vi "UHR-Fleezers Control (host) - 12.8.vi"() -> ()   [LabVIEW 2012] (continued)
              tunnel: w1167 -> [w1171]
              tunnel: w1166 -> [w1170]
              tunnel: w1165 -> [w1169]
              tunnel: w1164 -> [w1168]
              frame #0 {
                n826 = local write "BD 1 Frequency 1 (MHz)"(w1171) -> ()
                n827 = local write "BD 2 Frequency 1 (MHz)"(w1170) -> ()
                n828 = local write "BD 1 Frequency 2 (MHz)"(w1169) -> ()
                n829 = local write "BD 2 Frequency 2 (MHz)"(w1168) -> ()
              }
              frame #1 {
                n830 = property on="Update all trap values" class="Bool (strict)"("Val(Sgnl)"=TRUE ("Value (Signaling)")) -> ()  [unwired: 2 in, 2 out]
              }
            }
          }
        }
      }
      event "Stop All": Value Change {
        # "Stopping blue laser before shutting off program"
        n831 = event-data() -> ()  [unwired: 1 in, 5 out]
        n832 = local read "Delay (ms)"() -> (w1279:i32)
        n833 = call "serial write macro.vi"("String"="l0", "Delay (ms)"=w1279, "VISA resource name"=w1282) -> ("read buffer"=w1277:string, "error out"=w1278:errorcluster, "VISA resource name out"=w1281:refnum<visa-resource-name>)
        n834 = local write "read blue buffer"(w1277) -> ()
        n835 = local write "Blue Error Out"(w1278) -> ()
        n836 = VISA Close(VISA resource name=w1281) -> ()  [unwired: 1 in, 1 out]
        n837 = local read "Stop All"() -> (w1283:bool)
      }
    }
    n838 = node-c288() -> ()  [unwired: 1 in, 1 out]
  }
  n839 = node-c288(2 ("Processor")) -> (w66:T23)  [unwired: 3 out]
  n840 = node-c288() -> (w22:T23)  [unwired: 4 out]
  n841 = node-c288() -> (w68:T23)  [unwired: 4 out]
  n842 = while "Duncan's play event loop" {
    stop <- w1285 stop-if-true
    n843 = Create User Event(user event datatype=TRUE ("Boolean")) -> (user event=w1286:refnum<user-event>)  [unwired: 1 in, 1 out]
    n844 = Create User Event(user event datatype=TRUE ("Boolean")) -> (user event=w1293:refnum<user-event>)  [unwired: 1 in, 1 out]
    n845 = global write "Global for fluorescence simulation mean (30 samples), (power series).vi" "Red Signal"(w1286) -> ()
    n846 = global write "Global for fluorescence simulation mean (30 samples), (power series).vi" "Green Signal"(w1293) -> ()
    n847 = register-events(w1293, w1286) -> (reference out=w1292:refnum<event-registration>)  [unwired: 2 in, 1 out]
    n848 = event shown="[1] \"Get Fluorophore\": Value Change" {
      selector: w1292 -> [_ _ _ _]
      dyn-events: _ -> [_ _ _ _]
      timeout: 100 -> [_ _ _ _]
      event Timeout {
        n849 = event-data() -> ()  [unwired: 1 in, 2 out]
      }
      event "Get Fluorophore": Value Change {
        n850 = event-data() -> ("OldVal"=w1295:bool)  [unwired: 1 in, 4 out]
        n851 = case shown="True" w1295 {
          selector: w1295 -> [_ w1296]
          frame False {
          }
          frame True {
            n852 = property on="Move to Position 3" class="Bool"("Val(Sgnl)"=w1296) -> ()  [unwired: 2 in, 2 out]
            n853 = case shown="1" "Numeric" {
              frame 0, Default {
              }
              frame 1 {
                n854 = property on="Green Laser ON" class="Bool (strict)"("Val(Sgnl)"=TRUE ("Value (Signaling)")) -> ()  [unwired: 2 in, 2 out]
              }
              frame 2 {
                n855 = property on="Red Laser ON" class="Bool (strict)"("Val(Sgnl)"=TRUE) -> ()  [unwired: 2 in, 2 out]
              }
            }
          }
        }
      }
      event User Event {
        n856 = event-data() -> ("Boolean"=w1300:bool)  [unwired: 1 in, 3 out]
        "Green Fluorophore" <- w1300
        n857 = property on="Get Fluorophore" class="Bool (strict)"("Val(Sgnl)"=w1300) -> ()  [unwired: 2 in, 2 out]
      }
      event User Event {
        n858 = event-data() -> ("Boolean"=w1301:bool)  [unwired: 1 in, 3 out]
        "Red Fluorophore" <- w1301
        n859 = property on="Get Fluorophore" class="Bool (strict)"("Val(Sgnl)"=w1301) -> ()  [unwired: 2 in, 2 out]
      }
    }
    n860 = property on="Get Fluorophore" class="Bool (strict)"("Val(Sgnl)"="Get Fluorophore") -> ()  [unwired: 2 in, 2 out]
    n861 = Wait (ms)(milliseconds to wait=u32 100) -> ()  [unwired: 1 out]
    n862 = local read "Stop All"() -> (w1284:bool)
    n863 = Or(x=w1284, y="stop") -> (x .or. y?=w1285:bool)
  }
  n864 = timed-loop "Basic control parameters (all FPGA settings, other basic controls)" {
    shift-right: [w1309] -> _
    shift-left: errorcluster {"status"=FALSE, "code"=0, "source"=""} ("error out") -> [_]
    tunnel: [w1308] -> _
    timing: w66 -> [_]
    timing-out: [_] -> w65
    tunnel: w42 -> [w1307]
    tunnel: w32 -> [w1306]
    tunnel: w31 -> [w1305]
    tunnel: w30 -> [w1304]
    tunnel: w29 -> [w1303]
    tunnel: w5 -> [w1302]
    stop <- w1308 stop-if-true
    n865 = node-c288() -> ()  [unwired: 2 out]
    n866 = event shown="[35] \"+ phase (MCL)\", \"- phase (MCL)\": Value Change" {
      selector: _ -> [_ _ _ _ _ _ _ _ _ _ _ _ _ _ _ _ _ _ _ _ _ _ _ _ _ _ _ _ _ _ _ _ _ _ _ _ _ _ _ _ _ _ _ _ _ _ _ _ _ _ _ _ _ _ _ _ _ _ _ _ _ _ _ _ _ _ _ _ _ _ _ _ _ _]
      dyn-events: _ -> [_ _ _ _ _ _ _ _ _ _ _ _ _ _ _ _ _ _ _ _ _ _ _ _ _ _ _ _ _ _ _ _ _ _ _ _ _ _ _ _ _ _ _ _ _ _ _ _ _ _ _ _ _ _ _ _ _ _ _ _ _ _ _ _ _ _ _ _ _ _ _ _ _ _]
      timeout: _ -> [_ _ _ _ _ _ _ _ _ _ _ _ _ _ _ _ _ _ _ _ _ _ _ _ _ _ _ _ _ _ _ _ _ _ _ _ _ _ _ _ _ _ _ _ _ _ _ _ _ _ _ _ _ _ _ _ _ _ _ _ _ _ _ _ _ _ _ _ _ _ _ _ _ _]
      tunnel: [w1349 _ _ _ w1379 _ _ _ _ _ _ w1450 _ _ w1518 w1520 w1529 w1531 w1601 _ w1620 w1644 w1664 w1684 w1703 w1727 w1756 _ w1761 w1855 w1859 w1896 _ w1930 w1933 w1936 w1946 w1949 _ w1956 _ _ _ _ _ _ _ _ _ _ _ _ _ _ _ _ _ w2333 _ _ _ _ w2369 _ _ _ _ _ _ _ _ _ _ _] -> w1309
      tunnel: [_ _ _ _ _ _ _ _ _ w1435 _ _ _ _ _ _ _ _ _ _ _ _ _ _ _ _ _ _ _ _ _ _ _ _ _ _ _ _ _ _ _ _ _ _ _ _ _ _ _ _ _ _ _ _ _ _ _ _ _ _ _ _ _ _ _ _ _ _ _ _ _ _ _ _] -> w1308
      tunnel: [_ _ _ _ _ _ _ "Round T1 X" _ _ _ _ _ _ _ _ _ _ _ _ _ _ _ _ _ _ _ _ _ _ _ _ _ _ _ _ _ _ _ _ _ _ _ _ _ _ _ _ _ _ _ _ _ _ _ _ _ _ _ _ _ _ _ _ _ _ _ _ _ _ _ _ _ _] -> _
      tunnel: [_ _ _ "Adjust Scale\nto Mean" _ _ _ _ _ _ _ _ _ _ _ _ _ _ _ _ _ _ _ _ _ _ _ _ "Test ttrig" _ _ _ _ _ _ _ _ _ _ _ _ _ _ _ _ _ _ "Flush Sample" "Flush Pump 3" "Flush Pump 1" "Clear Volume" _ _ _ _ _ _ _ _ _ _ _ _ _ _ _ _ _ _ _ _ _ _ _] -> _
      tunnel: [_ _ _ _ _ _ _ _ "Round T2 X" _ "Delayed Interlace Start" _ _ _ _ _ _ _ _ _ _ _ _ _ _ _ _ _ _ _ _ _ _ _ _ _ _ _ _ _ _ _ _ _ _ _ _ _ _ _ _ _ _ _ _ _ _ _ _ _ _ _ _ _ _ _ _ _ _ _ _ _ _ _] -> _
      tunnel: w1307 -> [_ _ _ _ _ _ _ _ _ _ _ _ _ _ _ _ _ _ _ _ _ _ _ _ _ _ _ _ _ _ _ _ _ _ _ _ _ _ _ _ _ _ _ w2113 w2120 w2127 w2132 w2141 _ _ w2247 _ _ _ _ _ _ _ _ _ _ _ _ _ _ _ _ _ _ _ _ _ _ _]
      tunnel: w1306 -> [_ _ _ _ _ _ _ _ _ _ _ _ _ _ _ _ _ _ _ _ _ _ _ _ _ _ _ _ _ _ _ _ _ _ _ _ _ _ _ _ _ w2030 _ _ _ _ _ _ w2185 _ _ w2253 _ w2262 _ w2276 _ _ _ _ _ _ _ _ _ _ _ _ _ _ _ _ _ _]
      tunnel: w1305 -> [_ _ _ _ _ _ _ _ _ _ _ _ _ _ _ _ _ _ _ _ _ _ _ _ _ _ _ _ _ _ _ _ _ _ _ _ _ _ _ _ _ _ _ _ _ _ _ _ _ _ _ _ _ _ _ _ _ _ _ _ _ _ _ _ _ _ _ _ _ _ _ _ _ _]
      tunnel: w1304 -> [_ _ _ _ _ _ _ _ _ _ _ _ _ _ _ _ _ _ _ _ _ _ _ _ _ _ _ _ _ _ _ _ _ _ _ _ _ _ _ _ w1967 _ _ _ _ _ _ _ _ w2215 _ _ w2258 _ w2269 _ w2301 _ _ _ _ _ _ _ _ _ _ _ _ _ _ _ _ _]
      tunnel: w1303 -> [_ _ _ _ _ _ _ _ _ _ _ _ _ _ _ _ _ _ _ _ _ _ _ _ _ _ _ _ _ _ _ _ _ _ _ _ _ _ _ _ _ _ _ _ _ _ _ _ _ _ _ _ _ _ _ _ _ _ _ _ _ _ _ _ _ _ _ _ _ _ _ _ _ _]
      tunnel: w1302 -> [w1312 _ _ _ w1378 _ w1404 _ _ _ _ w1441 _ _ w1496 w1519 w1524 w1530 w1566 _ w1609 w1642 w1645 w1665 w1685 w1704 w1732 w1757 w1759 w1763 w1856 w1860 _ w1927 w1931 w1934 w1944 w1947 _ w1955 _ _ _ _ _ _ _ _ _ _ _ _ _ _ _ _ _ w2326 _ w2347 _ w2353 w2368 _ w2375 w2377 w2384 w2398 w2413 _ w2422 _ w2442 _]
      event "AI Count (ticks)", "Sets to FIFO (Traps)", "Save ave N", "FPGA Ave.", "# Samples/channel", "N sets to save": Value Change {
        # "So that if 'Save ave N' is updated, the AOD scanning code updates too."
        n867 = event-data() -> ()  [unwired: 6 out]
        n868 = local read "AI Count (ticks)"() -> (w1333:u16)
        n869 = Unbundle By Name("Sets to FIFO (Traps)") -> ("Set 1"=w1316:bool, "Set 2"=w1315:bool, "Set 3"=w1314:bool)
        n870 = Boolean To (0,1)(Boolean="Sets to FIFO (Traps)") -> (0, 1=w1341:cluster{"Set 1":i16, "Set 2":i16, "Set 3":i16})
        n871 = xnode "Read/Write Control"("FPGA VI Reference In"=w1312, "ai count"=w1333, "Set 1"=w1316, "Set 2"=w1315, "Set 3"=w1314, "N of AI1 Int Acq Sets"="N Acq Sets (Traps + Fl.)") -> ("error out"=w1349:errorcluster)  [unwired: 1 in, 1 out]
        n872 = Cluster To Array(cluster=w1341) -> (array=w1340:i16[])
        n873 = To Unsigned Long Integer(number=w1340) -> (unsigned 32bit integer=w1322:u32[])
        n874 = local read "Scan steps (AOD)"() -> (w1342:u64)
        n875 = Multiply(x=w1333, y="N Acq Sets (Traps + Fl.)") -> (x*y=w1331:u16)
        n876 = Divide(x=40000000.0, y=w1333) -> (x/y=w1325:dbl)
        "AI rate (Hz)" <- w1325
        "Ave. Rate (Hz)" <- w1325
        n877 = Add Array Elements(numeric array=w1322) -> (sum=w1334:u32)
        "Trap Sets" <- w1334
        n878 = Reciprocal(x=w1325) -> (1/x=→"Ave. Period (s)":dbl)
        n879 = property on="Scan steps (AOD)" class="DigNum (strict)"("Val(Sgnl)"=w1342) -> ()  [unwired: 2 in, 2 out]
        n880 = Divide(x=w1325, y="N Acq Sets (Traps + Fl.)") -> (x/y=w1346:dbl)
        "Data Rate (Hz)" <- w1346
        n881 = Reciprocal(x=w1346) -> (1/x=→"Data Period (s)":dbl)
        n882 = local read "Save ave N"() -> (w1345:dbl)
        n883 = Divide(x=w1346, y=w1345) -> (x/y=w1344:dbl)
        "Save Data Rate (Hz)" <- w1344
        n884 = Reciprocal(x=w1344) -> (1/x=→"Save Data Period (s)":dbl)
        n885 = Multiply(x=w1331, y="# Samples/trap") -> (x*y=w1329:u32)
        "Counts/DMA" <- w1329
        n886 = property on="Trap Disp. Downsample" class="DigNum (strict)"("Maximum"="# Samples/trap") -> ()  [unwired: 2 in, 2 out]
        n887 = Multiply(x=w1334, y="# Samples/trap") -> (x*y=w1323:u32)
        "# Samples/channel" <- w1323
        n888 = Multiply(x=w1323, y=u32 8) -> (x*y=→"Trap AI Elements/DMA read":u32)
        n889 = local read "APD Int. Count"() -> (w1330:u32)
        n890 = Multiply(x=w1323, y=u32 3) -> (x*y=→"Trap Pos Elements/DMA read":u32)
        n891 = Divide(x=w1329, y=w1330) -> (x/y=w1320:dbl)
        "APD Samples/FIFO Acq." <- w1320
        n892 = Divide(x=w1329, y=40000000.0) -> (x/y=w1327:dbl)
        "DMA Update Period (s)" <- w1327
        n893 = local read "Number of APDs"() -> (w1313:u8)
        n894 = Multiply(x=w1313, y=w1320) -> (x*y=→"APD Elements/DMA read":dbl)
        n895 = property on="APD Disp. Downsample" class="DigNum (strict)"("Maximum"=w1320) -> ()  [unwired: 2 in, 2 out]
        n896 = local read "N sets to save"() -> (w1339:u32)
        n897 = Multiply(x=w1327, y=w1339) -> (x*y=→"Total Time (s)":dbl)
        "FPGA Averaging" <- FALSE ("FPGA Averaging")
      }
      event "Remove Offset": Value Change {
        n898 = event-data() -> ()  [unwired: 7 out]
        n899 = local write "Remove Offset"(FALSE ("Remove Offset")) -> ()
        n900 = local read "Bead Mean (nm)"() -> (w1351:dbl)
        n901 = local read "Offset (nm)"() -> (w1352:dbl)
        n902 = Add(x=w1351, y=w1352) -> (x+y=w1350:dbl)
        n903 = local write "Offset (nm)"(w1350) -> ()
        n904 = disable-structure shown="Disabled" {
          frame Disabled {
            n905 = local read "Bead Mean (nm)"() -> (w1357:dbl)
            n906 = Add(y=w1357) -> (x=w1356:dbl, x+y=w1355:dbl)
            n907 = Subtract(x=w1357, y=w1356) -> (x-y=w1354:dbl)
            n908 = property on="Bead Separation" class="WFChart (strict)"("YScale.Minimum"=w1354) -> ()  [unwired: 2 in, 2 out]
            n909 = property on="Bead Separation" class="WFChart (strict)"("YScale.Maximum"=w1355) -> ()  [unwired: 2 in, 2 out]
          }
          frame Enabled {
          }
        }
      }
      event "Detector Type": Value Change {
        n910 = event-data() -> ()  [unwired: 7 out]
        n911 = local read "AI labels"() -> (w1359:string[])
        n912 = property on="High Res. Display" class="Ring (strict)"("Strings []"=w1359) -> ()  [unwired: 2 in, 2 out]
        n913 = Build Array (concatenate)(w1359, "none") -> (w1360:string[])
        n914 = property on="FFT 1 Choice 1" class="Ring (strict)"("Strings []"=w1360) -> ()  [unwired: 2 in, 2 out]
        n915 = property on="FFT 1 Choice 2" class="Ring (strict)"("Strings []"=w1360) -> ()  [unwired: 2 in, 2 out]
        n916 = property on="FFT 2 Choice 1" class="Ring (strict)"("Strings []"=w1360) -> ()  [unwired: 2 in, 2 out]
        n917 = property on="FFT 2 Choice 2" class="Ring (strict)"("Strings []"=w1360) -> ()  [unwired: 2 in, 2 out]
        n918 = Bundle("APD 1", "APD 2", "APD 3") -> (w1363:cluster{string, string, string})  [unwired: 1 out]
        n919 = Cluster To Array(cluster=w1363) -> (array=w1361:string[])
        n920 = Build Array (concatenate)(w1361, w1360) -> (w1365:string[])
        n921 = Array Size(array=w1365) -> (size(s)=w1366:i32)
        n922 = property on="Signals to Plot" class="LstBox (strict)"("Item Names"=w1365) -> ()  [unwired: 2 in, 2 out]
        n923 = property on="Signals to Plot" class="LstBox (strict)"("Number of Rows"=w1366) -> ()  [unwired: 2 in, 2 out]
        n924 = property on="All Signals" class="WFChart (strict)"("LegNumRows"=w1366) -> ()  [unwired: 2 in, 2 out]
      }
      event "Adjust Scale\nto Mean": Value Change {
        n925 = event-data() -> ()  [unwired: 7 out]
        n926 = local read "APD 1 Rate (Hz)"() -> (w1375:dbl)
        n927 = Multiply(x=1000.0, y="Above (kHz)") -> (x*y=w1373:dbl)
        n928 = Multiply(x=1000.0, y="Below (kHz)") -> (x*y=w1371:dbl)
        n929 = Add(x=w1373, y=w1375) -> (x+y=w1368:dbl)
        n930 = Subtract(x=w1375, y=w1371) -> (x-y=w1369:dbl)
        n931 = property on="APD Chart" class="WFChart (strict)"("YScale.Minimum"=w1369) -> ()  [unwired: 2 in, 2 out]
        n932 = property on="APD Chart" class="WFChart (strict)"("YScale.Maximum"=w1368) -> ()  [unwired: 2 in, 2 out]
      }
      event "Phase adj. (AI1)", "+ phase (AI1)", "- phase (AI1)": Value Change {
        n933 = event-data() -> ()  [unwired: 7 out]
        n934 = Negate(x="Phase adj. (AI1)") -> (-x=w1386:i16)
        n935 = Select(t=w1386, s="- phase (AI1)", f="Phase adj. (AI1)") -> (s? t:f=w1385:i16)
        n936 = xnode "Read/Write Control"("FPGA VI Reference In"=w1378, "Phase count adjustment"=w1385) -> ("FPGA VI Reference Out"=w1384:T20, "error out"=w1383:errorcluster)  [unwired: 2 in]
        n937 = Or(x="- phase (AI1)", y="+ phase (AI1)") -> (x .or. y?=w1380:bool)
        n938 = xnode "Read/Write Control"("FPGA VI Reference In"=w1384, "error in"=w1383, "+ phase"=w1380) -> ("error out"=w1379:errorcluster)  [unwired: 1 in, 1 out]
      }
      event "Signals to Plot": Double Click {
        w1390 = u32 9868950 ("Color Box")
        n939 = event-data() -> ("Row"=w1392:i32)  [unwired: 9 out]
        n940 = property on="All Signals" class="WFChart (strict)"("Active Plot"=w1392) -> (error out=w1403:errorcluster)  [unwired: 2 in, 1 out]
        n941 = property on="All Signals" class="WFChart (strict)" props=["Plot", "Visible?", "Plot", "Plot Color"](error in=w1403) -> (error out=w1402:errorcluster, "Plot.Visible?"=w1401:bool)  [unwired: 1 in, 2 out]
        n942 = Select(t=FALSE ("Plot.Visible"), s=w1401, f=TRUE ("Plot.Visible")) -> (s? t:f=w1396:bool)
        n943 = property on="All Signals" class="WFChart (strict)"(error in=w1402, "Plot.Visible?"=w1396) -> (error out=w1398:errorcluster)  [unwired: 1 in, 1 out]
        n944 = property on="All Signals" class="WFChart (strict)"(error in=w1398) -> (error out=w1393:errorcluster, "Plot.Plot Color"=w1397:u32)  [unwired: 1 in, 1 out]
        n945 = property on="Signals to Plot" class="LstBox (strict)"(error in=w1393, "Active Row"=w1392) -> (error out=w1391:errorcluster)  [unwired: 1 in, 1 out]
        n946 = Select(t=w1397, s=w1396, f=u32 0) -> (s? t:f=w1394:u32)
        n947 = property on="Signals to Plot" class="LstBox (strict)"(error in=w1391, "CellFontColor"=w1394, "SelColor"=w1390, "CellBG"=w1390, "CellFontSize"=u32 20 ("Active Row:Cell Font:Size"), "CellFontBold"=TRUE ("Active Row:Cell Font:Bold")) -> ()  [unwired: 1 in, 2 out]
      }
      event "BD 1 Frequency 1 (MHz)", "BD 1 Frequency 2 (MHz)", "BD 1 Frequency 3 (MHz)", "BD 2 Frequency 1 (MHz)", "BD 2 Frequency 2 (MHz)", "BD 2 Frequency 3 (MHz)", "Trap Delta (MHz)", "Update all trap values": Value Change {
        # "This is so you can set trap frequencies\nvia local variables and then update\nall at once"
        n948 = event-data() -> ("CtlRef"=w1408:refnum<vi>)  [unwired: 6 out]
        n949 = control-ref of="Trap Delta (MHz)"() -> (w1407:refnum<vi>)
        n950 = Equal?(x=w1407, y=w1408) -> (x = y?=w1406:bool)
        n951 = local write "Update all trap values"(FALSE ("Update all trap values")) -> ()
        n952 = case shown="False" "Oscillate Set 1" {
          tunnel: w1406 -> [w1412 _]
          tunnel: w1404 -> [w1410 _]
          frame False {
            n953 = local read "BD 1 Frequency 2 (MHz)"() -> (w1416:dbl)
            n954 = local read "BD 1 Frequency 1 (MHz)"() -> (w1414:dbl)
            n955 = Subtract(x=w1416, y="Trap Delta (MHz)") -> (x-y=w1413:dbl)
            n956 = Select(t=w1413, s=w1412, f=w1414) -> (s? t:f=w1411:dbl)
            n957 = local read "Y RF Frequency Limits (MHz)"() -> (w1417:T16)
            n958 = local read "X RF Frequency Limits (MHz)"() -> (w1418:T16)
            n959 = local write "BD 1 Frequency 1 (MHz)"(w1411) -> ()
            n960 = local read "BD 1 Frequency 3 (MHz)"() -> (w1427:dbl)
            n961 = local read "BD 2 Frequency 1 (MHz)"() -> (w1421:dbl)
            n962 = local read "BD 2 Frequency 2 (MHz)"() -> (w1420:dbl)
            n963 = local read "BD 2 Frequency 3 (MHz)"() -> (w1428:dbl)
            n964 = call "set RF board frequency - interlace.vi"("Board 2 Frequency Limits"=w1417, "Board 1 Frequency Limits"=w1418, "FPGA VI Reference In"=w1410, "Board 2 Frequency 3 (MHz)"=w1428, "Board 1 Frequency 3 (MHz)"=w1427, "Board 2 Frequency 2 (MHz)"=w1420, "Board 2 Frequency 1 (MHz)"=w1421, "Board 1 Frequency 2 (MHz)"=w1416, "Board 1 Frequency 1  (MHz)"=w1411) -> ()  [unwired: 1 in, 2 out]
            n965 = Subtract(x=w1421, y=w1420) -> (x-y=w1425:dbl)
            n966 = Subtract(x=w1411, y=w1416) -> (x-y=w1426:dbl)
            n967 = Square(x=w1425) -> (x^2=w1423:dbl)
            n968 = Square(x=w1426) -> (x^2=w1424:dbl)
            n969 = Add(x=w1424, y=w1423) -> (x+y=w1422:dbl)
            n970 = Square Root(x=w1422) -> (sqrt(x)=w1419:dbl)
            n971 = property on="Initial delta (MHz)" class="DigNum (strict)"("Val(Sgnl)"=w1419) -> ()  [unwired: 2 in, 2 out]
            n972 = local write "Trap Delta (MHz)"(w1419) -> ()
          }
          frame True {
          }
        }
      }
      event "Round T1 X": Value Change {
        n973 = event-data() -> ()  [unwired: 7 out]
        n974 = local read "BD 1 Frequency 1 (MHz)"() -> (w1431:dbl)
        n975 = Round To Nearest(number=w1431) -> (nearest integer value=w1430:dbl)
        n976 = property on="BD 1 Frequency 1 (MHz)" class="DigNum (strict)"("Val(Sgnl)"=w1430) -> ()  [unwired: 2 in, 2 out]
      }
      event "Round T2 X": Value Change {
        n977 = event-data() -> ()  [unwired: 7 out]
        n978 = local read "BD 1 Frequency 2 (MHz)"() -> (w1433:dbl)
        n979 = Round To Nearest(number=w1433) -> (nearest integer value=w1432:dbl)
        n980 = property on="BD 1 Frequency 2 (MHz)" class="DigNum (strict)"("Val(Sgnl)"=w1432) -> ()  [unwired: 2 in, 2 out]
      }
      event "Stop All": Value Change {
        n981 = event-data() -> ()  [unwired: 7 out]
        n982 = local read "Stop All"() -> (w1435:bool)
      }
      event "Delayed Interlace Start": Value Change {
        n983 = event-data() -> ()  [unwired: 7 out]
        n984 = flat-sequence {
          frame #0 {
            n985 = Multiply(x="Delay to Interlace (s)", y=1000.0) -> (x*y=w1437:dbl)
            n986 = Wait (ms)(milliseconds to wait=w1437) -> ()  [unwired: 1 out]
          }
          frame #1 {
            n987 = property on="Laser interlacing mode" class="RadioBtnsControl (strict)"("Val(Sgnl)"=enum32{"Laser ON", "Laser OFF", "Interlace"}."Interlace" ("Value (Signaling)")) -> ()  [unwired: 2 in, 2 out]
          }
        }
      }
      event "BD 1 Amplitude 1 (%)", "BD 1 Amplitude 2 (%)", "BD 1 Amplitude 3 (%)", "BD 2 Amplitude 1 (%)", "BD 2 Amplitude 2 (%)", "BD 2 Amplitude 3 (%)", "Trap 1 ON", "Trap 2 ON", "Trap 3 ON", "Feedback On/Off", "All FB On/Off": Value Change {
        w1462 = i16 1 ("f")
        n988 = event-data() -> ()  [unwired: 7 out]
        n989 = local write "Trap 1 (ON/OFF)"("Trap 1 ON") -> ()
        n990 = local write "Trap 2 (ON/OFF)"("Trap 2 ON") -> ()
        n991 = Boolean To (0,1)(Boolean="Trap 3 ON") -> (0, 1=w1463:i16)
        n992 = Boolean To (0,1)(Boolean="Trap 1 ON") -> (0, 1=w1464:i16)
        n993 = Boolean To (0,1)(Boolean="Trap 2 ON") -> (0, 1=w1465:i16)
        n994 = Select(t=w1465, s="Trap ON/OFF X or Y Amp?", f=w1462) -> (s? t:f=w1460:i16)
        n995 = Select(t=w1464, s="Trap ON/OFF X or Y Amp?", f=w1462) -> (s? t:f=w1461:i16)
        n996 = Select(t=w1463, s="Trap ON/OFF X or Y Amp?", f=w1462) -> (s? t:f=w1459:i16)
        n997 = Select(t=w1462, s="Trap ON/OFF X or Y Amp?", f=w1465) -> (s? t:f=w1457:i16)
        n998 = Select(t=w1462, s="Trap ON/OFF X or Y Amp?", f=w1464) -> (s? t:f=w1458:i16)
        n999 = Select(t=w1462, s="Trap ON/OFF X or Y Amp?", f=w1463) -> (s? t:f=w1456:i16)
        n1000 = And(x="All FB On/Off", y="Feedback On/Off") -> (x .and. y?=w1454:cluster{"Set 1":bool, "Set 2":bool})
        n1001 = local read "BD 1 Amplitude 1 (%)"() -> (w1472:dbl)
        n1002 = local read "BD 1 Amplitude 2 (%)"() -> (w1471:dbl)
        n1003 = local read "BD 1 Amplitude 3 (%)"() -> (w1470:dbl)
        n1004 = Unbundle By Name(w1454) -> ("Set 1"=w1449:bool, "Set 2"=w1446:bool)
        n1005 = local read "Y RF Amplitude Limits (%)"() -> (w1442:T16)
        n1006 = local read "X RF Amplitude Limits (%)"() -> (w1443:T16)
        n1007 = local read "BD 2 Amplitude 1 (%)"() -> (w1473:dbl)
        n1008 = local read "BD 2 Amplitude 2 (%)"() -> (w1474:dbl)
        n1009 = local read "BD 2 Amplitude 3 (%)"() -> (w1475:dbl)
        n1010 = And(x="Trap 2 ON", y=w1446) -> (x .and. y?=w1444:bool)
        n1011 = And(x="Trap 1 ON", y=w1449) -> (x .and. y?=w1447:bool)
        n1012 = Multiply(x=w1461, y=w1472) -> (x*y=w1469:dbl)
        n1013 = Multiply(x=w1471, y=w1460) -> (x*y=w1467:dbl)
        n1014 = Multiply(x=w1470, y=w1459) -> (x*y=w1468:dbl)
        n1015 = Multiply(x=w1473, y=w1458) -> (x*y=w1476:dbl)
        n1016 = Multiply(x=w1474, y=w1457) -> (x*y=w1477:dbl)
        n1017 = Multiply(x=w1475, y=w1456) -> (x*y=w1478:dbl)
        n1018 = call "set RF board amplitude - interlace.vi"("Board 2 Amplitude Limits"=w1442, "Board 1 Amplitude Limits"=w1443, "FPGA VI Reference In"=w1441, "Board 2 Amplitude 3 (%)"=w1478, "Board 1 Amplitude 3 (%)"=w1468, "Board 2 Amplitude 2 (%)"=w1477, "Board 2 Amplitude 1 (%)"=w1476, "Board 1 Amplitude 2 (%)"=w1467, "Board 1 Amplitude 1 (%)"=w1469) -> ("error out"=w1451:errorcluster, "FPGA VI Reference Out"=w1452:T20)  [unwired: 1 in]
        n1019 = xnode "Read/Write Control"("FPGA VI Reference In"=w1452, "error in"=w1451, "FB On/Off Set 1"=w1447, "FB On/Off Set 2"=w1444) -> ("error out"=w1450:errorcluster)  [unwired: 1 out]
      }
      event "Load parameters": Value Change {
        n1020 = event-data() -> ()  [unwired: 7 out]
        n1021 = property on="Saved AOD Raster Scan Parameter Sets" class="Arr (strict)"() -> ("Index Values"=w1489:u32[])  [unwired: 2 in, 2 out]
        n1022 = Index Array(array=w1489, index=0) -> (element=w1486:u32)
        n1023 = local write "Load parameters"(FALSE ("Load parameters")) -> ()
        n1024 = Index Array(array="Saved AOD Raster Scan Parameter Sets", index=w1486) -> (element=w1485:T30)
        n1025 = Unbundle By Name(w1485) -> ("Scan Range AOD (nm) 2"=w1484:dbl, "Step Size AOD (nm) 2"=w1483:dbl, "Scan Speed AOD (nm/s) 2"=w1482:dbl, "Number of scans (AOD) 2"=w1481:u16)
        n1026 = flat-sequence {
          tunnel: w1484 -> [w1492]
          tunnel: w1483 -> [w1491]
          tunnel: w1482 -> [w1490]
          tunnel: w1481 -> [w1493]
          frame #0 {
            n1027 = local write "Scan Speed (nm/s)"(w1490) -> ()
            n1028 = local write "Scan Range (nm)"(w1492) -> ()
            n1029 = local write "Step Size (nm)"(w1491) -> ()
          }
          frame #1 {
            n1030 = property on="Number of F/B Scans (AOD)" class="DigNum (strict)"("Val(Sgnl)"=w1493) -> ()  [unwired: 2 in, 2 out]
          }
        }
      }
      event "Trap 1 (ON/OFF)", "Trap 2 (ON/OFF)": Value Change {
        n1031 = event-data() -> ()  [unwired: 7 out]
        n1032 = property on="Trap 2 ON" class="Bool (strict)"("Val(Sgnl)"="Trap 2 (ON/OFF)") -> ()  [unwired: 2 in, 2 out]
        n1033 = property on="Trap 1 ON" class="Bool (strict)"("Val(Sgnl)"="Trap 1 (ON/OFF)") -> ()  [unwired: 2 in, 2 out]
      }
      event "DIO count 1 (ticks)", "DIO count 2 (ticks)", "DIO count 3 (ticks)", "Interlace", "Number Interlace Sets", "Not-Interlacing Set", "BD 1 Delay (ticks)", "BD 2 Delay (Ticks)", "Next trap write delay (ticks)", "XY phase ext loop method", "Amp switch delay 2", "BD 2 Delay (Ticks) 2", "BD 1 Delay (ticks) 2": Value Change {
        n1034 = event-data() -> ()  [unwired: 7 out]
        n1035 = local read "DIO count 3 (ticks)"() -> (w1514:u16)
        n1036 = local read "DIO count 1 (ticks)"() -> (w1516:u16)
        n1037 = local read "DIO count 2 (ticks)"() -> (w1515:u16)
        n1038 = To Unsigned Byte Integer(number="Not-Interlacing Set") -> (unsigned 8bit integer=w1505:u8)
        n1039 = Add(x=w1505, y=u8 1) -> (x+y=w1509:u8)
        n1040 = xnode "Read/Write Control"("FPGA VI Reference In"=w1496, "DIO count 1 (ticks)"=w1516, "DIO count 2 (ticks)"=w1515, "DIO count 3 (ticks)"=w1514, "Interlace ON/OFF"="Interlace", "Number Interlace Cycles"="Number Interlace Sets", "Interlace Off Parameters"=w1509, "BD 1 Delay (ticks)"="BD 1 Delay (ticks)", "BD 2 Delay (Ticks)"="BD 2 Delay (Ticks)", "Next trap write delay (ticks)"="Next trap write delay (ticks)", "XY phase ext loop method"="XY phase ext loop method", "Amp switch delay 2"="Amp switch delay 2", "BD 2 Delay (Ticks) 2"="BD 2 Delay (Ticks) 2", "BD 1 Delay (ticks) 2"="BD 1 Delay (ticks) 2") -> ("error out"=w1518:errorcluster)  [unwired: 1 in, 1 out]
        n1041 = Build Array(w1516, w1515, w1514) -> (w1507:u16[])
        n1042 = Split 1D Array(array=w1507, index="Number Interlace Sets") -> (first subarray=w1517:u16[])  [unwired: 1 out]
        n1043 = Index Array(array=w1507, index=w1505) -> (element=w1506:u16)
        n1044 = Add Array Elements(numeric array=w1517) -> (sum=w1511:u16)
        n1045 = Select(t=w1511, s="Interlace", f=w1506) -> (s? t:f=→"Total Counts (ticks)":u16)
      }
      event "Reset Feedback": Value Change {
        n1046 = event-data() -> ()  [unwired: 7 out]
        n1047 = Unbundle By Name("Reset Feedback") -> ("Set 1"=w1522:bool, "Set 2"=w1521:bool)
        n1048 = xnode "Read/Write Control"("FPGA VI Reference In"=w1519, "FB Reset Set 1"=w1522, "FB Reset Set 2"=w1521) -> ("error out"=w1520:errorcluster)  [unwired: 1 in, 1 out]
      }
      event "Trap Intensity PID Gains": Value Change {
        n1049 = event-data() -> ()  [unwired: 7 out]
        n1050 = Unbundle By Name("Trap Intensity PID Gains") -> ("proportional gain (Kc)"=w1527:i16, "integral gain (Kc*Ts/Ti)"=w1526:i16, "derivative gain (Kc*Td/Ts)"=w1525:i16)
        n1051 = xnode "Read/Write Control"("FPGA VI Reference In"=w1524, "P1"=w1527, "I1"=w1526, "D1"=w1525) -> ("error out"=w1529:errorcluster)  [unwired: 1 in, 1 out]
      }
      event "AI2 to Setpoint", "Setpoints (V)": Value Change {
        n1052 = event-data() -> ()  [unwired: 7 out]
        n1053 = xnode "Read/Write Control"("FPGA VI Reference In"=w1530) -> ("FPGA VI Reference Out"=w1533:T20, "error out"=w1532:errorcluster, "AI2 Y Sum Set 1"=w1540:i16, "AI2 Y Sum Set 2"=w1539:i16)  [unwired: 1 in]
        n1054 = Cluster To Array(cluster="AI2 to Setpoint") -> (array=w1543:bool[])
        n1055 = local read "AI2 (V)"() -> (w1541:cluster{"Set 1":dbl, "Set 2":dbl})
        n1056 = Or Array Elements(Boolean array=w1543) -> (logical OR=w1544:bool)
        n1057 = Bundle By Name(cluster=w1541, "Set 1"=w1540, "Set 2"=w1539) -> (w1538:cluster{"Set 1":dbl, "Set 2":dbl})
        n1058 = Divide(x=w1538, y=3276.7) -> (x/y=w1537:cluster{"Set 1":dbl, "Set 2":dbl})
        "AI2 (V)" <- w1537
        n1059 = case shown="True" w1544 {
          tunnel: [w1547 w1564] -> w1536
          tunnel: "AI2 to Setpoint" -> [_ w1560]
          tunnel: "Setpoints (V)" -> [w1548 w1563]
          tunnel: w1537 -> [_ w1557]
          frame False {
            n1060 = Multiply(x=3276.7, y=w1548) -> (x*y=w1549:cluster{"Set 1":dbl, "Set 2":dbl})
            n1061 = To Word Integer(number=w1549) -> (16bit integer=w1547:cluster{"Set 1":i16, "Set 2":i16})
          }
          frame True {
            n1062 = Unbundle By Name(w1557) -> ("Set 1"=w1556:dbl, "Set 2"=w1555:dbl)
            n1063 = Unbundle By Name(w1563) -> ("Set 1"=w1562:dbl, "Set 2"=w1561:dbl)
            n1064 = Unbundle By Name(w1560) -> ("Set 1"=w1559:bool, "Set 2"=w1558:bool)
            n1065 = Select(t=w1556, s=w1559, f=w1562) -> (s? t:f=w1554:dbl)
            n1066 = Select(t=w1555, s=w1558, f=w1561) -> (s? t:f=w1553:dbl)
            n1067 = Bundle By Name(cluster=w1563, "Set 1"=w1554, "Set 2"=w1553) -> (w1551:cluster{"Set 1":dbl, "Set 2":dbl})
            n1068 = local write "Setpoints (V)"(w1551) -> ()
            n1069 = Multiply(x=3276.7, y=w1551) -> (x*y=w1552:cluster{"Set 1":dbl, "Set 2":dbl})
            n1070 = To Word Integer(number=w1552) -> (16bit integer=w1564:cluster{"Set 1":i16, "Set 2":i16})
          }
        }
        n1071 = Unbundle By Name(w1536) -> ("Set 1"=w1535:i16, "Set 2"=w1534:i16)
        n1072 = xnode "Read/Write Control"("FPGA VI Reference In"=w1533, "error in"=w1532, "FB Setpoint Set 1"=w1535, "FB Setpoint Set 2"=w1534) -> ("error out"=w1531:errorcluster)  [unwired: 1 out]
      }
      event "+ phase (GI)", "- phase (GI)", "+ phase (GI) 2", "- phase (GI) 2", "+ phase (RI)", "- phase (RI)", "+ phase (Green FB)", "- phase (Green FB)": Value Change {
        n1073 = event-data() -> ()  [unwired: 7 out]
        n1074 = Or(x="+ phase (GI)", y="- phase (GI)") -> (x .or. y?=w1600:bool)
        n1075 = Negate(x="Phase adj. (GI)") -> (-x=w1605:i16)
        n1076 = Select(t=w1605, s="+ phase (GI)", f="Phase adj. (GI)") -> (s? t:f=w1604:i16)
        n1077 = Or(x="+ phase (GI) 2", y="- phase (GI) 2") -> (x .or. y?=w1591:bool)
        n1078 = Negate(x="Phase adj. (GI) 2") -> (-x=w1596:i16)
        n1079 = Select(t=w1596, s="+ phase (GI) 2", f="Phase adj. (GI) 2") -> (s? t:f=w1592:i16)
        n1080 = Negate(x="Phase adj. (RI)") -> (-x=w1590:i16)
        n1081 = Or(x="+ phase (RI)", y="- phase (RI)") -> (x .or. y?=w1586:bool)
        n1082 = Select(t=w1590, s="+ phase (RI)", f="Phase adj. (RI)") -> (s? t:f=w1585:i16)
        n1083 = Or(x="+ phase (Green FB)", y="- phase (Green FB)") -> (x .or. y?=w1579:bool)
        n1084 = Negate(x="Phase adj. (Green FB)") -> (-x=w1584:i16)
        n1085 = Select(t=w1584, s="+ phase (Green FB)", f="Phase adj. (Green FB)") -> (s? t:f=w1580:i16)
        n1086 = Negate(x="Phase adj. (BI AO)") -> (-x=w1578:i16)
        n1087 = Or(x="+ phase (BI AO)", y="- phase (BI AO)") -> (x .or. y?=w1568:bool)
        n1088 = Select(t=w1578, s="+ phase (BI AO)", f="Phase adj. (BI AO)") -> (s? t:f=w1570:i16)
        n1089 = Negate(x="Phase adj. (BI DO)") -> (-x=w1574:i16)
        n1090 = Or(x="+ phase (BI DO)", y="- phase (BI DO)") -> (x .or. y?=w1567:bool)
        n1091 = Select(t=w1574, s="+ phase (BI DO)", f="Phase adj. (BI DO)") -> (s? t:f=w1569:i16)
        n1092 = xnode "Read/Write Control"("FPGA VI Reference In"=w1566, "Phase count adjustment (GI)"=w1604, "Phase count adjustment (GI) 2"=w1592, "Phase count adjustment (RI)"=w1585, "Phase count adjustment (Green FB)"=w1580, "Phase count adjustment (BI AO)"=w1570, "Phase count adjustment (BI D)"=w1569) -> ("FPGA VI Reference Out"=w1602:T20, "error out"=w1603:errorcluster)  [unwired: 1 in]
        n1093 = xnode "Read/Write Control"("FPGA VI Reference In"=w1602, "error in"=w1603, "+ phase (GI)"=w1600, "+ phase (GI) 2"=w1591, "+ phase (RI)"=w1586, "+ phase (Green FB)"=w1579, "+ phase (BI AO)"=w1568, "+ phase (BI D)"=w1567) -> ("error out"=w1601:errorcluster)  [unwired: 1 out]
      }
      event "Green Laser ON/OFF", "Red Laser ON/OFF", "Blue Laser ON/OFF": Value Change {
        # "This loop shouldn't be initialized.  The main 'laser ON' settings should dominate and set the others."
        n1094 = event-data() -> ()  [unwired: 7 out]
        n1095 = property on="Red Laser ON" class="Bool (strict)"("Val(Sgnl)"="Red Laser ON/OFF") -> ()  [unwired: 2 in, 2 out]
        n1096 = property on="Blue Laser ON" class="Bool (strict)"("Val(Sgnl)"="Blue Laser ON/OFF") -> ()  [unwired: 2 in, 2 out]
        n1097 = property on="Green Laser ON" class="Bool (strict)"("Val(Sgnl)"="Green Laser ON/OFF") -> ()  [unwired: 2 in, 2 out]
      }
      event "Laser interlacing mode", "Green Laser ON", "Red Laser ON", "Blue Laser ON": Value Change {
        n1098 = event-data() -> ()  [unwired: 7 out]
        n1099 = local write "Green Laser ON/OFF"("Green Laser ON") -> ()
        n1100 = local write "Blue Laser ON/OFF"("Blue Laser ON") -> ()
        n1101 = local write "Red Laser ON/OFF"("Red Laser ON") -> ()
        n1102 = case shown="True" "Green Laser ON" {
          tunnel: "Laser interlacing mode" -> [_ w1641]
          tunnel: [enum32{"Laser ON", "Laser OFF", "Interlace"}."Laser OFF" ("Green laser mode") w1641] -> w1619
          tunnel: [FALSE w1637] -> w1618
          frame False {
          }
          frame True {
            n1103 = local read "Green FB On/Off"() -> (w1638:bool)
            n1104 = Equal?(x=w1641, y=enum32{"Laser ON", "Laser OFF", "Interlace"}."Interlace") -> (x = y?=w1639:bool)
            n1105 = And(x=w1639, y=w1638) -> (x .and. y?=w1637:bool)
          }
        }
        n1106 = case shown="True" "Red Laser ON" {
          tunnel: "Laser interlacing mode" -> [_ w1634]
          tunnel: [enum32{"Laser ON", "Laser OFF", "Interlace"}."Laser OFF" ("Green laser mode") w1634] -> w1615
          tunnel: [FALSE w1630] -> w1614
          frame False {
          }
          frame True {
            n1107 = local read "Red FB On/Off"() -> (w1631:bool)
            n1108 = Equal?(x=w1634, y=enum32{"Laser ON", "Laser OFF", "Interlace"}."Interlace") -> (x = y?=w1632:bool)
            n1109 = And(x=w1632, y=w1631) -> (x .and. y?=w1630:bool)
          }
        }
        n1110 = case shown="True" "Blue Laser ON" {
          tunnel: "Laser interlacing mode" -> [_ w1625]
          tunnel: [enum32{"Laser ON", "Laser OFF", "Interlace"}."Laser OFF" ("Green laser mode") w1625] -> w1611
          tunnel: [FALSE w1623] -> w1610
          frame False {
          }
          frame True {
            n1111 = local read "Blue FB On/Off"() -> (w1624:bool)
            n1112 = Equal?(x=w1625, y=enum32{"Laser ON", "Laser OFF", "Interlace"}."Interlace") -> (x = y?=w1626:bool)
            n1113 = And(x=w1626, y=w1624) -> (x .and. y?=w1623:bool)
          }
        }
        n1114 = xnode "Read/Write Control"("FPGA VI Reference In"=w1609, "Operating Mode"=w1619, "Operating Mode 2"=w1619, "Green FB On/Off"=w1618, "Red Laser Operating Mode"=w1615, "RI Operating Mode 2"=w1615, "Red FB On/Off"=w1614, "BI Operating Mode (AO)"=w1611, "Blue Laser Operating Mode (D)"=w1611, "Blue FB On/Off"=w1610) -> ("error out"=w1620:errorcluster)  [unwired: 1 in, 1 out]
      }
      event "Invert laser interlacing": Value Change {
        n1115 = event-data() -> ()  [unwired: 7 out]
        n1116 = xnode "Read/Write Control"("FPGA VI Reference In"=w1642, "Invert GI"="Invert laser interlacing", "Invert GI 2"="Invert laser interlacing", "Invert RI"="Invert laser interlacing", "Invert RI 2"="Invert laser interlacing", "Invert BI (AO)"="Invert laser interlacing", "Invert BI (D)"="Invert laser interlacing") -> ("error out"=w1644:errorcluster)  [unwired: 1 in, 1 out]
      }
      event "Green FB Setpoint (mV)", "Green FB Gains", "Green FB On/Off", "Green Intensity % (FB OFF)", "Green int current ON count adj": Value Change {
        n1117 = event-data() -> ()  [unwired: 7 out]
        n1118 = local read "Green FB Setpoint (mV)"() -> (w1656:dbl)
        n1119 = Multiply(x=w1656, y=3.2767) -> (x*y=w1655:dbl)
        n1120 = local read "Green Intensity % (FB OFF)"() -> (w1659:dbl)
        n1121 = Multiply(x=w1659, y=655.35) -> (x*y=w1660:dbl)
        n1122 = To Unsigned Word Integer(number=w1660) -> (unsigned 16bit integer=w1658:u16)
        n1123 = local read "Green int current ON count adj"() -> (w1662:u32)
        n1124 = local read "Laser interlacing mode"() -> (w1652:enum32{"Laser ON", "Laser OFF", "Interlace"})
        n1125 = local read "Green FB Gains"() -> (w1649:T9)
        n1126 = local read "Green Laser ON"() -> (w1653:bool)
        n1127 = local read "Green FB On/Off"() -> (w1663:bool)
        n1128 = Equal?(x=w1652, y=enum32{"Laser ON", "Laser OFF", "Interlace"}."Interlace") -> (x = y?=w1650:bool)
        n1129 = Unbundle By Name(w1649) -> ("proportional gain (Kc)"=w1648:i16, "integral gain (Kc*Ts/Ti)"=w1647:i16, "derivative gain (Kc*Td/Ts)"=w1646:i16)
        n1130 = Compound Arithmetic op=AND(w1650, w1663, w1653) -> (w1654:bool)
        n1131 = xnode "Read/Write Control"("FPGA VI Reference In"=w1645, "Green FB Setpoint"=w1655, "Green FB On/Off"=w1654, "Current Out"=w1658, "Green int current ON count adj"=w1662, "P3"=w1648, "I3"=w1647, "D3"=w1646) -> ("error out"=w1664:errorcluster)  [unwired: 1 in, 1 out]
      }
      event "Blue FB Setpoint (mV)", "Blue FB Gains", "Blue FB On/Off", "Blue Intensity % (FB OFF)", "Blue int AO ON count adjust": Value Change {
        # "16 bit analog out"
        n1132 = event-data() -> ()  [unwired: 7 out]
        n1133 = Multiply(x="Blue FB Setpoint (mV)", y=3.2767) -> (x*y=w1679:dbl)
        n1134 = Multiply(x="Blue Intensity % (FB OFF)", y=655.35) -> (x*y=w1682:dbl)
        n1135 = To Unsigned Word Integer(number=w1682) -> (unsigned 16bit integer=w1681:u16)
        n1136 = local read "Laser interlacing mode"() -> (w1677:enum32{"Laser ON", "Laser OFF", "Interlace"})
        n1137 = Unbundle By Name("Blue FB Gains") -> ("proportional gain (Kc)"=w1674:i16, "integral gain (Kc*Ts/Ti)"=w1673:i16, "derivative gain (Kc*Td/Ts)"=w1672:i16)
        n1138 = local read "Blue Laser ON"() -> (w1666:bool)
        n1139 = Equal?(x=w1677, y=enum32{"Laser ON", "Laser OFF", "Interlace"}."Interlace") -> (x = y?=w1675:bool)
        n1140 = Compound Arithmetic op=AND(w1675, "Blue FB On/Off", w1666) -> (w1678:bool)
        n1141 = xnode "Read/Write Control"("FPGA VI Reference In"=w1665, "Blue FB Setpoint"=w1679, "Blue FB On/Off"=w1678, "BI Current Out"=w1681, "Blue current ON count adj (AO)"="Blue int AO ON count adjust", "P5"=w1674, "I5"=w1673, "D5"=w1672) -> ("error out"=w1684:errorcluster)  [unwired: 1 in, 1 out]
      }
      event "Red FB Setpoint (mV)", "Red FB Gains", "Red FB On/Off", "Red Intensity % (FB OFF)": Value Change {
        n1142 = event-data() -> ()  [unwired: 7 out]
        n1143 = local read "Red FB Setpoint (mV)"() -> (w1697:dbl)
        n1144 = Multiply(x=w1697, y=3.2767) -> (x*y=w1696:dbl)
        n1145 = local read "Red Intensity % (FB OFF)"() -> (w1686:dbl)
        n1146 = Multiply(x=w1686, y=655.35) -> (x*y=w1700:dbl)
        n1147 = To Unsigned Word Integer(number=w1700) -> (unsigned 16bit integer=w1699:u16)
        n1148 = local read "Laser interlacing mode"() -> (w1693:enum32{"Laser ON", "Laser OFF", "Interlace"})
        n1149 = local read "Red FB Gains"() -> (w1690:T9)
        n1150 = local read "Red Laser ON"() -> (w1694:bool)
        n1151 = local read "Red FB On/Off"() -> (w1702:bool)
        n1152 = Equal?(x=w1693, y=enum32{"Laser ON", "Laser OFF", "Interlace"}."Interlace") -> (x = y?=w1691:bool)
        n1153 = Unbundle By Name(w1690) -> ("proportional gain (Kc)"=w1689:i16, "integral gain (Kc*Ts/Ti)"=w1688:i16, "derivative gain (Kc*Td/Ts)"=w1687:i16)
        n1154 = Compound Arithmetic op=AND(w1691, w1702, w1694) -> (w1695:bool)
        n1155 = xnode "Read/Write Control"("FPGA VI Reference In"=w1685, "Red FB Setpoint"=w1696, "Red FB On/Off"=w1695, "RI Current Out"=w1699, "P4"=w1689, "I4"=w1688, "D4"=w1687) -> ("error out"=w1703:errorcluster)  [unwired: 1 in, 1 out]
      }
      event "+ phase (APD 1 Gate)", "- phase (APD 1 Gate)", "+ phase (APD 2 Gate)", "- phase (APD 2 Gate)", "+ phase (APD 3 Gate)", "- phase (APD 3 Gate)", "+ phase (APD Acq)", "- phase (APD Acq)": Value Change {
        n1156 = event-data() -> ()  [unwired: 7 out]
        n1157 = local read "Phase Adj. (APD 1 Gate)"() -> (w1724:i16)
        n1158 = Or(x="- phase (APD 1 Gate)", y="+ phase (APD 1 Gate)") -> (x .or. y?=w1726:bool)
        n1159 = Negate(x=w1724) -> (-x=w1731:i16)
        n1160 = Select(t=w1731, s="+ phase (APD 1 Gate)", f=w1724) -> (s? t:f=w1730:i16)
        n1161 = local read "Phase Adj. (APD 2 Gate)"() -> (w1721:i16)
        n1162 = Or(x="- phase (APD 2 Gate)", y="+ phase (APD 2 Gate)") -> (x .or. y?=w1719:bool)
        n1163 = Negate(x=w1721) -> (-x=w1723:i16)
        n1164 = Select(t=w1723, s="+ phase (APD 2 Gate)", f=w1721) -> (s? t:f=w1720:i16)
        n1165 = Negate(x="Phase Adj. (APD 3 Gate)") -> (-x=w1718:i16)
        n1166 = Or(x="- phase (APD 3 Gate)", y="+ phase (APD 3 Gate)") -> (x .or. y?=w1714:bool)
        n1167 = Select(t=w1718, s="+ phase (APD 3 Gate)", f="Phase Adj. (APD 3 Gate)") -> (s? t:f=w1715:i16)
        n1168 = local read "Phase Adj. (APD Acq)"() -> (w1712:i16)
        n1169 = Or(x="- phase (APD Acq)", y="+ phase (APD Acq)") -> (x .or. y?=w1710:bool)
        n1170 = Negate(x=w1712) -> (-x=w1713:i16)
        n1171 = Select(t=w1713, s="+ phase (APD Acq)", f=w1712) -> (s? t:f=w1711:i16)
        n1172 = xnode "Read/Write Control"("FPGA VI Reference In"=w1704, "Phase count adjustment (APD 1 Gate)"=w1730, "Phase count adjustment (APD 2 Gate)"=w1720, "Phase count adjustment (APD 3 Gate)"=w1715, "Phase Count Adjustment (APD Acq)"=w1711) -> ("FPGA VI Reference Out"=w1728:T20, "error out"=w1729:errorcluster)  [unwired: 1 in]
        n1173 = xnode "Read/Write Control"("FPGA VI Reference In"=w1728, "error in"=w1729, "+ phase (APD 1 Gate)"=w1726, "+ phase (APD 2 Gate)"=w1719, "+ phase (APD 3 Gate)"=w1714, "+ phase (APD Acq)"=w1710) -> ("error out"=w1727:errorcluster)  [unwired: 1 out]
      }
      event "Invert APD Gate", "APD Gate ON Count", "APD Gate OFF Count", "APD Gate", "APD Integration Time (s)", "APD AO Scale Factor", "Duty Frequency (ON 1/N cycles)", "Interlace ON count", "Interlace OFF count": Value Change {
        n1174 = event-data() -> ()  [unwired: 7 out]
        n1175 = Add(x="Interlace ON count", y="Interlace OFF count") -> (x+y=w1738:u16)
        n1176 = Add(x="APD Gate ON Count", y="APD Gate OFF Count") -> (x+y=w1749:u16)
        n1177 = Multiply(x="Duty Frequency (ON 1/N cycles)", y=w1738) -> (x*y=w1734:u16)
        "Green AI Count" <- w1734
        "Red AI Count" <- w1734
        "Blue AI Count" <- w1734
        n1178 = Subtract(x=w1734, y="Interlace ON count") -> (x-y=w1737:u16)
        n1179 = Multiply(x=w1749, y="Duty Frequency (ON 1/N cycles)") -> (x*y=w1748:u16)
        n1180 = Subtract(x=w1748, y="APD Gate ON Count") -> (x-y=w1747:u16)
        n1181 = local read "DMA Update Period (s)"() -> (w1750:dbl)
        n1182 = Multiply(x="APD Integration Time (s)", y=40000000.0) -> (x*y=w1754:dbl)
        n1183 = Reciprocal(x="APD Integration Time (s)") -> (1/x=→"APD Acq Rate (Hz)":dbl)
        n1184 = To Unsigned Long Integer(number=w1754) -> (unsigned 32bit integer=w1740:u32)
        "APD Int. Count" <- w1740
        n1185 = local read "Number of APDs"() -> (w1733:u8)
        n1186 = Divide(x=w1750, y="APD Integration Time (s)") -> (x/y=w1752:dbl)
        n1187 = Multiply(x=w1733, y=w1752) -> (x*y=w1751:dbl)
        n1188 = local write "APD Samples/FIFO Acq."(w1752) -> ()
        n1189 = local write "APD Elements/DMA read"(w1751) -> ()
        n1190 = xnode "Read/Write Control"("FPGA VI Reference In"=w1732, "Invert APD Gate"="Invert APD Gate", "APD Gate ON Count"="APD Gate ON Count", "APD Gate OFF Count"=w1747, "APD Acq Rate Count"=w1740, "APD Gate Operating Mode"="APD Gate", "APD AO scale factor"="APD AO Scale Factor", "Green interlace ON count"="Interlace ON count", "Green interlace OFF count"=w1737, "Green interlace ON count 2"="Interlace ON count", "Green interlace OFF count 2"=w1737, "Green FB Count"=w1734, "Red interlace ON count"="Interlace ON count", "Red interlace OFF count"="Interlace OFF count", "Blue ON count (AO)"="Interlace ON count", "Blue OFF count (AO)"="Interlace OFF count", "Blue interlace OFF count (D)"="Interlace OFF count", "Blue interlace ON count (D)"="Interlace ON count") -> ("error out"=w1756:errorcluster)  [unwired: 1 in, 1 out]
      }
      event "Neg. TTrig FPGA": Value Change {
        n1191 = event-data() -> ()  [unwired: 7 out]
        n1192 = xnode "Read/Write Control"("FPGA VI Reference In"=w1757, "TTrig Negate Pos"="Neg. TTrig FPGA") -> ()  [unwired: 1 in, 2 out]
      }
      event "Test ttrig": Value Change {
        n1193 = event-data() -> ()  [unwired: 7 out]
        n1194 = xnode "Read/Write Control"("FPGA VI Reference In"=w1759, "TTrig?"=TRUE) -> ("error out"=w1761:errorcluster)  [unwired: 1 in, 1 out]
      }
      event "Number of F/B Scans (AOD)", "Scan Speed (nm/s)", "Scan BD", "Initial delta (MHz)", "Step Size (nm)", "Scan Range (nm)": Value Change {
        w1825 = 123.0  # AOM cal (nm/MHz)
        n1195 = event-data() -> ()  [unwired: 7 out]
        n1196 = local read "BD 1 Frequency 1 (MHz)"() -> (w1808:dbl)
        n1197 = local read "AOM X Cal (nm/MHz)"() -> (w1800:dbl)
        n1198 = local read "X RF Frequency Limits (MHz)"() -> (w1812:T16)
        n1199 = local read "Y RF Frequency Limits (MHz)"() -> (w1809:T16)
        n1200 = local read "BD 2 Frequency 1 (MHz)"() -> (w1814:dbl)
        n1201 = Negate(x="Scan Range (nm)") -> (-x=w1778:dbl)
        n1202 = Divide(x=w1778, y=w1800) -> (x/y=w1782:dbl)
        n1203 = Select(t=w1812, s="Scan BD", f=w1809) -> (s? t:f=w1811:T16)
        n1204 = Select(t=w1808, s="Scan BD", f=w1814) -> (s? t:f=w1813:dbl)
        n1205 = Unbundle By Name(w1811) -> ("Maximum"=w1820:dbl, "Minimum"=w1819:dbl)
        n1206 = Add(x=w1782, y=w1813) -> (x+y=w1817:dbl)
        n1207 = Divide(x=w1778, y="Step Size (nm)") -> (x/y=w1797:dbl)
        n1208 = Divide(x="Step Size (nm)", y=w1800) -> (x/y=w1806:dbl)
        n1209 = Absolute Value(x=w1797) -> (abs(x)=w1781:dbl)
        n1210 = Sign(1:w1778) -> (0:w1779:dbl)
        n1211 = In Range and Coerce(upper limit=w1820, x=w1817, lower limit=w1819) -> (coerced(x)=w1816:dbl, In Range?=w1818:bool)
        n1212 = To Unsigned Quad Integer(1:w1781) -> (0:w1796:u64)
        "Scan steps (AOD)" <- w1796
        n1213 = call "IR AOM freq to word.vi"("Frequency In (MHz)"=w1806) -> ("Frequency Word Out (double)"=w1803:dbl)
        n1214 = Multiply(x=w1779, y=w1803) -> (x*y=w1780:dbl)
        n1215 = Subtract(x=w1817, y=w1816) -> (x-y=w1815:dbl)
        n1216 = To Quad Integer(1:w1780) -> (0:w1802:i64)
        "Incr. int (AOD)" <- w1802
        n1217 = Subtract(x=w1782, y=w1815) -> (x-y=w1801:dbl)
        "Scan Range (MHz)" <- w1801
        n1218 = Select(t=w1782, s=w1818, f=w1801) -> (s? t:f=w1821:dbl)
        n1219 = Multiply(x=w1801, y=w1800) -> (x*y=w1799:dbl)
        n1220 = Decrement(x=w1796) -> (x-1=w1849:u64)
        n1221 = Negate(x=w1799) -> (-x=w1795:dbl)
        n1222 = local write "Scan Range (nm)"(w1795) -> ()
        n1223 = Divide(x=w1821, y=w1849) -> (x/y=w1805:dbl)
        "Scan Increment (MHz)" <- w1805
        n1224 = call "IR AOM freq to word.vi"("Frequency In (MHz)"=w1805) -> ("Frequency Word Out (double)"=w1804:dbl)
        n1225 = Divide(x="Step Size (nm)", y="Scan Speed (nm/s)") -> (x/y=w1792:dbl)
        n1226 = To Quad Integer(1:w1804) -> ()  [unwired: 1 out]
        n1227 = local read "Number Interlace Sets"() -> (w1776:u8)
        n1228 = local read "AI Count (ticks)"() -> (w1777:u16)
        n1229 = local read "Total Counts (ticks)"() -> (w1775:u16)
        n1230 = local read "# Samples/trap"() -> (w1807:u32)
        n1231 = Multiply(x=w1777, y=w1776) -> (x*y=w1774:u16)
        n1232 = Divide(x=w1775, y=w1774) -> (x/y=w1773:dbl)
        n1233 = Select(t=w1808, s="Scan BD", f=w1814) -> (s? t:f=w1846:dbl)
        "Initial freq. (MHz)" <- w1846
        n1234 = Add(x=w1821, y=w1846) -> (x+y=→"Final freq. (MHz)":dbl)
        n1235 = Divide(x=w1775, y=40000000.0) -> (x/y=w1791:dbl)
        n1236 = Divide(x=w1792, y=w1791) -> (x/y=w1790:dbl)
        n1237 = To Unsigned Quad Integer(1:w1790) -> (0:w1765:u64)
        n1238 = Quotient & Remainder(x=w1765, y=u64 2) -> (x-y*floor(x/y)=w1769:u64)  [unwired: 1 out]
        n1239 = Equal?(x=w1769, y=u64 0) -> (x = y?=w1767:bool)
        n1240 = Decrement(x=w1765) -> (x-1=w1766:u64)
        n1241 = Select(t=w1765, s=w1767, f=w1766) -> (s? t:f=w1764:u64)
        "Cycles/step (AOD)" <- w1764
        n1242 = xnode "Read/Write Control"("FPGA VI Reference In"=w1763, "Scan steps"=w1796, "Number of scans"="Number of F/B Scans (AOD)", "Cycles per step"=w1764, "Scan freq.  increment"=w1802, "Scan BD"="Scan BD") -> ("error out"=w1855:errorcluster)  [unwired: 1 in, 1 out]
        n1243 = Multiply(x=w1796, y=w1764) -> (x*y=w1850:u64)
        n1244 = Multiply(x=w1850, y=u64 2) -> (x*y=w1772:u64)
        n1245 = Multiply(x=w1773, y=w1772) -> (x*y=w1771:dbl)
        "Data points/scan (f/b)" <- w1771
        n1246 = Multiply(x=w1771, y="Number of F/B Scans (AOD)") -> (x*y=w1853:dbl)
        "Data points/scans" <- w1853
        n1247 = Divide(x=w1853, y=w1807) -> (x/y=→"N sets should be saved":dbl)
        n1248 = Multiply(x=w1850, y=w1791) -> (x*y=w1789:dbl)
        "Time/Scan (s) (AOD)" <- w1789
        n1249 = Select(t=w1821, s="Scan BD", f=0.0) -> (s? t:f=w1847:dbl)
        n1250 = Select(t=0.0, s="Scan BD", f=w1821) -> (s? t:f=w1843:dbl)
        n1251 = local read "BD 2 Frequency 2 (MHz)"() -> (w1839:dbl)
        n1252 = local read "BD 1 Frequency 2 (MHz)"() -> (w1842:dbl)
        n1253 = Add(x=w1843, y=w1814) -> (x+y=w1840:dbl)
        n1254 = Add(x=w1808, y=w1847) -> (x+y=w1841:dbl)
        n1255 = Multiply(x=w1789, y=2.0) -> (x*y=w1788:dbl)
        n1256 = Multiply(x=w1788, y="Number of F/B Scans (AOD)") -> (x*y=w1785:dbl)
        n1257 = Divide(x=w1785, y=60.0) -> (x/y=→"Time to Finish All (min)":dbl)
        n1258 = Add(x="Trap 2 Bead Size (nm)", y="Trap 1 Bead Size (nm)") -> (x+y=w1829:dbl)
        n1259 = Divide(x=w1829, y=2.0) -> (x/y=w1823:dbl)
        n1260 = local read "Initial delta (MHz)"() -> (w1826:dbl)
        n1261 = Subtract(x=w1840, y=w1839) -> (x-y=w1837:dbl)
        n1262 = Subtract(x=w1841, y=w1842) -> (x-y=w1838:dbl)
        n1263 = Square(x=w1837) -> (x^2=w1836:dbl)
        n1264 = Square(x=w1838) -> (x^2=w1835:dbl)
        n1265 = Add(x=w1835, y=w1836) -> (x+y=w1834:dbl)
        n1266 = Square Root(x=w1834) -> (sqrt(x)=w1833:dbl)
        "Final delta (MHz)" <- w1833
        n1267 = Multiply(x=w1825, y=w1833) -> (x*y=w1832:dbl)
        n1268 = Multiply(x=w1826, y=w1825) -> (x*y=w1824:dbl)
        n1269 = Subtract(x=w1824, y=w1823) -> (x-y=→"Initial sep (nm)":dbl)
        n1270 = Subtract(x=w1832, y=w1823) -> (x-y=→"Final sep (nm)":dbl)
      }
      event "Freq or Amp switch first", "Swap F1 and F2", "Freq switch delay", "Amp switch delay": Value Change {
        n1271 = event-data() -> ()  [unwired: 7 out]
        n1272 = local read "Amp switch delay"() -> (w1857:u16)
        n1273 = local read "Swap F1 and F2"() -> (w1858:bool)
        n1274 = xnode "Read/Write Control"("FPGA VI Reference In"=w1856, "Swap F1 and F2"=w1858, "Amp switch delay"=w1857) -> ("error out"=w1859:errorcluster)  [unwired: 1 in, 1 out]
      }
      event "Scan steps (MCL)", "Number of scans (MCL)", "Scan Range (V)\n(of steps)", "2D or 1D Scan", "N APD Samp/step", "Fast Scan Dir", "Continuous MCL Scanning", "Scan lines (y)": Value Change {
        w1862 = 32767.0 ("y")
        n1275 = event-data() -> ()  [unwired: 7 out]
        n1276 = Select(t="Scan lines (y)", s="2D or 1D Scan", f="Number of scans (MCL)") -> (s? t:f=w1867:u64)
        n1277 = Decrement(x="Scan steps (MCL)") -> (x-1=w1883:u64)
        n1278 = Divide(x="Scan Range (V)\n(of steps)", y=w1883) -> (x/y=w1882:dbl)
        "Desired Scan Incr (V)" <- w1882
        n1279 = local read "APD Integration Time (s)"() -> (w1875:dbl)
        n1280 = Multiply(x=w1882, y=w1862) -> (x*y=w1891:dbl)
        n1281 = Divide(x=w1891, y=10.0) -> (x/y=w1881:dbl)
        "Desired incr (int)" <- w1881
        n1282 = local read "Update Count (MCL)"() -> (w1887:u32)
        n1283 = Round Toward -Infinity(1:w1881) -> (0:w1890:dbl)
        n1284 = To Word Integer(number=w1890) -> (16bit integer=w1865:i16)
        "Actual Incr. int (MCL)" <- w1865
        n1285 = Multiply(x=w1875, y=40000000.0) -> (x*y=w1888:dbl)
        n1286 = Divide(x=w1888, y=w1887) -> (x/y=w1886:dbl)
        n1287 = Multiply(x=i16 10, y=w1865) -> (x*y=w1863:i16)
        n1288 = Multiply(x="N APD Samp/step", y=w1886) -> (x*y=w1885:dbl)
        "Cycles/step (MCL)" <- w1885
        n1289 = Divide(x=w1863, y=w1862) -> (x/y=→"Actual MCL Inc (V)":dbl)
        n1290 = Multiply(x="N APD Samp/step", y="Scan steps (MCL)") -> (x*y=w1877:dbl)
        n1291 = local read "APD Samples/FIFO Acq."() -> (w1874:dbl)
        n1292 = Multiply(x=w1877, y=u64 2) -> (x*y=w1876:dbl)
        "Data points/scan (f+b)" <- w1876
        n1293 = Multiply(x=w1876, y=w1867) -> (x*y=w1894:dbl)
        "Data points/scans (MCL)" <- w1894
        n1294 = Multiply(x=w1875, y=w1876) -> (x*y=w1868:dbl)